vi "UHR-Fleezers Control (host) - Avogadro v2.vi"() -> ()   [LabVIEW 2014] (continued)
      tunnel: w4863 -> [w5493 w5511]
      tunnel: w4862 -> [w5492 w5510]
      tunnel: [w5493 w5506] -> w4814
      tunnel: [w5492 w5505] -> w4813
      tunnel: [FALSE w5504] -> w4846
      tunnel: "Start MCL Scan" -> [_ w5501]
      tunnel: "Confocal Image" -> [_ w5500]
      tunnel: "Confocal Linescan" -> [_ _]
      frame False {
      }
      frame True {
        w5504 = TRUE
        n3101 = case shown="True" "Restart DMA? (MCL)" {
          tunnel: [w5587 w5589] -> w5509
          tunnel: [w5586 w5588] -> w5508
          tunnel: w5511 -> [w5587 w5592]
          tunnel: w5510 -> [w5586 w5591]
          frame False {
          }
          frame True {
            n3102 = call "reset FPGA DMA.vi"("error in"=w5591, "FPGA VI Reference In"=w5592) -> ("error out"=w5588:errorcluster, "FPGA VI Reference Out"=w5589:T40)
            n3103 = local write "Overflow (data lost)"(FALSE ("Overflow (data lost)")) -> ()
          }
        }
        n3104 = case shown="False" w5501 {
          tunnel: w5500 -> [w5514 _]
          frame False {
            n3105 = property on="Confocal Image" class="Bool (strict)"("Value"=FALSE ("Start Confocal Map")) -> ()  [unwired: 2 in, 2 out]
            n3106 = property on="2D or 1D Scan" class="Bool (strict)"("Val(Sgnl)"=w5514) -> ()  [unwired: 2 in, 2 out]
          }
          frame True {
          }
        }
        n3107 = local write "Tab Control 6"(T62."Imaging" ("Tab Control 6")) -> ()
        n3108 = local read "T3 X (V)"() -> (w5496:dbl)
        n3109 = local write "MCL Scanning"(w5504) -> ()
        n3110 = local read "T3 Y (V)"() -> (w5495:dbl)
        n3111 = local read "AO2"() -> (w5497:dbl)
        n3112 = local read "AO1"() -> (w5498:dbl)
        n3113 = case shown="True" "Center Scan" {
          tunnel: w5509 -> [w5527 w5549]
          tunnel: w5508 -> [w5526 w5548]
          tunnel: [w5525 w5547] -> w5506
          tunnel: [w5524 w5546] -> w5505
          tunnel: [w5519 w5543] -> w5503
          tunnel: [w5520 w5542] -> w5502
          tunnel: w5498 -> [w5517 w5545]
          tunnel: w5497 -> [w5516 w5544]
          tunnel: "Scan trap 3 or Fl?" -> [w5522 w5541]
          tunnel: w5496 -> [w5521 w5534]
          tunnel: w5495 -> [w5518 w5535]
          frame False {
            w5523 = TRUE ("AI to FIFO")
            n3114 = case shown="False" w5522 {
              tunnel: [w5529 w5533] -> w5520
              tunnel: w5521 -> [_ w5533]
              tunnel: [w5530 w5532] -> w5519
              tunnel: w5518 -> [_ w5532]
              tunnel: w5517 -> [w5530 _]
              tunnel: w5516 -> [w5529 _]
              tunnel: [FALSE ("AI to FIFO") TRUE ("AI to FIFO")] -> w5515
              frame False {
              }
              frame True {
              }
            }
            n3115 = xnode "Read/Write Control"("FPGA VI Reference In"=w5527, "error in"=w5526, "AI to FIFO"=w5523, "APD to FIFO"=w5523, "Start scan (MCL)"=w5523, "ScanTrap 3 or Fl-laser"=w5515) -> ("FPGA VI Reference Out"=w5525:T40, "error out"=w5524:errorcluster)
          }
          frame True {
            n3116 = local read "Actual MCL Inc (V)"() -> (w5536:dbl)
            n3117 = local read "Scan steps (MCL)"() -> (w5537:u64)
            n3118 = local read "Scan lines (y)"() -> (w5538:u64)
            n3119 = local read "Fast Scan Dir"() -> (w5539:bool)
            n3120 = local read "2D or 1D Scan"() -> (w5540:bool)
            n3121 = case shown="False" w5541 {
              tunnel: w5549 -> [w5567 w5585]
              tunnel: w5548 -> [w5566 w5584]
              tunnel: [w5565 w5583] -> w5547
              tunnel: [w5564 w5582] -> w5546
              tunnel: w5545 -> [w5560 _]
              tunnel: w5544 -> [w5559 _]
              tunnel: [w5557 w5577] -> w5543
              tunnel: [w5556 w5576] -> w5542
              tunnel: w5540 -> [w5555 w5575]
              tunnel: w5539 -> [w5554 w5574]
              tunnel: w5538 -> [w5553 w5573]
              tunnel: w5537 -> [w5552 w5572]
              tunnel: w5536 -> [w5550 w5570]
              tunnel: w5535 -> [_ w5569]
              tunnel: w5534 -> [_ w5568]
              frame False {
                w5563 = TRUE ("AI to FIFO")
                n3122 = Bundle("Actual MCL Inc (V)"=w5550, "Scan steps (MCL)"=w5552, "Scan lines (y)"=w5553, "AO1"=w5560, "AO2"=w5559) -> (w5558:T66)  [unwired: 1 in]
                n3123 = call "Center Scan calculation.vi"("2D or 1D Scan"=w5555, "Fast Scan Dir"=w5554, "Input parameters"=w5558) -> ("X"=w5556:dbl, "Y"=w5557:dbl)
                n3124 = call "Volt to I16.vi"("Voltage In"=w5557) -> ("I16 Voltage Out"=w5562:i16)
                n3125 = call "Volt to I16.vi"("Voltage In"=w5556) -> ("I16 Voltage Out"=w5561:i16)
                n3126 = xnode "Read/Write Control"("FPGA VI Reference In"=w5567, "error in"=w5566, "AI to FIFO"=w5563, "APD to FIFO"=w5563, "Start scan (MCL)"=w5563, "AO1 (Y)"=w5562, "AO2 (X)"=w5561, "ScanTrap 3 or Fl-laser"=FALSE ("AI to FIFO")) -> ("FPGA VI Reference Out"=w5565:T40, "error out"=w5564:errorcluster)
              }
              frame True {
                w5581 = TRUE ("AI to FIFO")
                n3127 = Bundle("Actual MCL Inc (V)"=w5570, "Scan steps (MCL)"=w5572, "Scan lines (y)"=w5573, "T3 Y (V)"=w5569, "T3 X (V)"=w5568) -> (w5578:T67)  [unwired: 1 in]
                n3128 = call "Center Scan calculation.vi"("2D or 1D Scan"=w5575, "Fast Scan Dir"=w5574, "Input parameters"=w5578) -> ("X"=w5576:dbl, "Y"=w5577:dbl)
                n3129 = call "Volt to I16.vi"("Voltage In"=w5577) -> ("I16 Voltage Out"=w5580:i16)
                n3130 = call "Volt to I16.vi"("Voltage In"=w5576) -> ("I16 Voltage Out"=w5579:i16)
                n3131 = xnode "Read/Write Control"("FPGA VI Reference In"=w5585, "error in"=w5584, "AI to FIFO"=w5581, "APD to FIFO"=w5581, "Start scan (MCL)"=w5581, "Piezo Trap Y (AO4)"=w5580, "Piezo Trap X (AO5)"=w5579, "ScanTrap 3 or Fl-laser"=TRUE ("AI to FIFO")) -> ("FPGA VI Reference Out"=w5583:T40, "error out"=w5582:errorcluster)
              }
            }
          }
        }
        "Initial Y" <- w5503
        "Initial X" <- w5502
        "wait to reset values" <- w5504
      }
    }
    n3132 = xnode "Read/Write Control"("FPGA VI Reference In"=w4675) -> ("FPGA VI Reference Out"=w4570:T40, "BD1 Frequency Out 1"=w4677:u64, "Piezo X out"=w4609:i16, "Piezo Y out"=w4608:i16)  [unwired: 1 in, 1 out]
    n3133 = And(x="Save scans", y=w4843) -> (x .and. y?=w4861:bool)
    n3134 = call "IR AOM word to freq.vi"("Frequency Word In (U64)"=w4677) -> ("Frequency Out (MHz)"=w4676:dbl)
    n3135 = Divide(x=w4609, y=w4643) -> (x/y=w4642:dbl)
    n3136 = Divide(x=w4608, y=w4643) -> (x/y=w4641:dbl)
    n3137 = local read "BD 1 Frequency 2 (MHz)"() -> (w4707:dbl)
    n3138 = Subtract(x=w4707, y=w4676) -> (x-y=w4640:dbl)
    "Current deltaF (MHz)" <- w4640
    n3139 = Build Array(w4640, w4642, w4641) -> (w4566:dbl[])
    "Trap position array" <- w4566
    n3140 = control-ref of="Piezo trap cursor control"() -> (w4649:refnum<vi>)
    n3141 = Unbundle By Name("Cursor control") -> ("X"=w4651:bool, "Y"=w4650:bool)
    n3142 = local read "APD Elements/DMA read"() -> (w4738:u32)
    n3143 = local read "Trap AI Elements/DMA read"() -> (w4835:u32)
    n3144 = case shown="False" w4651 {
      tunnel: w4649 -> [w4998 w5008]
      tunnel: w4570 -> [_ w5000]
      frame False {
        n3145 = local read "T3 X (V)"() -> (w4999:dbl)
        n3146 = property class="XYGraph (strict)"(reference=w4998, "Cursor.Cursor X"=w4999) -> ()  [unwired: 1 in, 2 out]
      }
      frame True {
        n3147 = property class="XYGraph (strict)"(reference=w5008) -> ("Cursor.Cursor X"=w5005:dbl)  [unwired: 1 in, 2 out]
        n3148 = In Range and Coerce(upper limit=10.0, x=w5005, lower limit=0.0) -> (coerced(x)=w5003:dbl)  [unwired: 1 out]
        n3149 = Multiply(x=3276.7, y=w5003) -> (x*y=w5002:dbl)
        n3150 = To Unsigned Word Integer(number=w5002) -> (unsigned 16bit integer=w5001:u16)
        n3151 = xnode "Read/Write Control"("FPGA VI Reference In"=w5000, "Piezo Trap X (AO5)"=w5001) -> ()  [unwired: 1 in, 2 out]
      }
    }
    n3152 = case shown="False" w4650 {
      tunnel: w4649 -> [w4985 w4997]
      tunnel: w4570 -> [_ w4988]
      frame False {
        n3153 = local read "T3 Y (V)"() -> (w4987:dbl)
        n3154 = Negate(x=w4987) -> (-x=w4986:dbl)
        n3155 = property class="XYGraph (strict)"(reference=w4985, "Cursor.Cursor Y"=w4986) -> ()  [unwired: 1 in, 2 out]
      }
      frame True {
        n3156 = property class="XYGraph (strict)"(reference=w4997) -> ("Cursor.Cursor Y"=w4994:dbl)  [unwired: 1 in, 2 out]
        n3157 = In Range and Coerce(upper limit=0.0, x=w4994, lower limit=-10.0) -> (coerced(x)=w4993:dbl)  [unwired: 1 out]
        n3158 = Negate(x=w4993) -> (-x=w4991:dbl)
        n3159 = Multiply(x=3276.7, y=w4991) -> (x*y=w4990:dbl)
        n3160 = To Unsigned Word Integer(number=w4990) -> (unsigned 16bit integer=w4989:u16)
        n3161 = xnode "Read/Write Control"("FPGA VI Reference In"=w4988, "Piezo Trap Y (AO4)"=w4989) -> ()  [unwired: 1 in, 2 out]
      }
    }
    n3162 = local read "Trap Pos Elements/DMA read"() -> (w4810:u32)
    n3163 = local read "DMA Update Period (s)"() -> (w4691:dbl)
    n3164 = xnode "Invoke Method"("FPGA VI Reference In"=w4814, "error in"=w4813, "Number of Elements"=w4810, "Timeout (ms)"=-1) -> ("Data"=w4646:u16[], "Elements Remaining"=→"Trap Pos FIFO El Remaining":u32)  [unwired: 2 out]
    n3165 = xnode "Get Trap Data"("FPGA VI Reference In"=w4814, "error in"=w4813, "Number of Elements"=w4835, "Timeout (ms)"=-1 ("Timeout")) -> ("FPGA VI Reference Out"=w4706:T40, "error out"=w4762:errorcluster, "Data"=w4695:i16[], "Elements Remaining"=w4895:u32)
    "FIFO El. Rem." <- w4895
    n3166 = local read "Trap AI FIFO Depth"() -> (w4897:u32)
    n3167 = xnode "Get APD Data"("FPGA VI Reference In"=w4814, "error in"=w4813, "Number of Elements"=w4738, "Timeout (ms)"=-1) -> ("Data"=w4687:u32[], "Elements Remaining"=→"APD FIFO Elements Remaining":u32)  [unwired: 2 out]
    n3168 = feedback #1(0.0) -> (w4808:dbl)
    n3169 = To Time Stamp(1:w4808) -> (0:w4590:timestamp)
    n3170 = Add(x=w4691, y=w4808) -> (x+y=w4872:dbl)
    n3171 = feedback-in #1(w4872) -> ()
    n3172 = Subtract(x=w4897, y=w4835) -> (x-y=w4896:u32)
    n3173 = local read "APD Integration Time (s)"() -> (w4679:dbl)
    n3174 = Divide(x=w4895, y=w4896) -> (x/y=w4894:dbl)
    "Buffer Status" <- w4894
    n3175 = local read "Trap Sets"() -> (w4696:u32)
    n3176 = Equal?(x=w4894, y=1.0) -> (x = y?=w4892:bool)
    n3177 = local read "Number of APDs"() -> (w4686:u8)
    n3178 = case "Alert buffer overflow" shown="True" w4892 {
      frame False {
      }
      frame True {
        n3179 = call <vilib>:"Beep.vi"() -> ()  [unwired: 3 in, 9 out]
        "Overflow (data lost)" <- TRUE ("Overflow (data lost)")
      }
    }
    n3180 = call "deinterlace.vi"("Detector type"="Detector Type", "Data"=w4695, "Trap sets"=w4696, "Flip x sign"="Flip X Sign") -> ("Channel pattern"=w4692:i32, "Channel names"=w4648:string[], "Deinterlaced normalized data"=w4584:dbl[][], "Deinterlaced data"=w4693:i16[])
    "AI labels" <- w4648
    n3181 = local read "Data Period (s)"() -> (w4583:dbl)
    n3182 = call "Trap_position_vectors.vi"("Data array"=w4646) -> ("Output data for plotting"=w4645:dbl[][], "Output data for saving"=w4644:u64[])
    n3183 = call "APD data extraction.vi"("Data"=w4687, "Number of APD's"=w4686, "APD integration time (s)"=w4679, "APD Ave N"="APD Ave N", "APD Disp. Downsample"="APD Disp. Downsample", "APD Disp. Scale"="APD Disp. Scale", "Time Stamp"=w4590) -> ("Output cluster"=→"APD rates cluster":T2, "Output Data"=w4682:T68, "Output waveform"=w4681:waveform(dbl)[], "APD Display period (s)"=w4680:dbl)
    "APD Display Period (s)" <- w4680
    n3184 = Reciprocal(x=w4680) -> (1/x=→"APD Display Freq. (Hz)":dbl)
    n3185 = Multiply(x=w4583, y="Trap Disp. Downsample") -> (x*y=w4809:dbl)
    "Display Period (s)" <- w4809
    n3186 = for {
      tunnel: w4584 -> [w5023] mode=indexing
      tunnel: [w5022] -> w4647 mode=indexing
      n3187 = call-poly <vilib>:"Mean.vi"("X"=w5023) -> ("mean"=w5022:dbl)  [unwired: 1 out]
    }
    "Values" <- w4647
    n3188 = Decimate 1D Array(w4693) -> (w4800:i16[], w4799:i16[], w4797:i16[], w4796:i16[])  [unwired: 9 out]
    n3189 = call "Generate Waveform.vi"("Downsampling"="Trap Disp. Downsample", "Data Period (s)"=w4583, "Data"=w4584, "Plot names"=w4648, "Time Stamp"=w4590) -> ("Downsampled data"=w4626:waveform(dbl)[], "Non downsampled waveform"=w4688:waveform(dbl)[])
    n3190 = Multiply(x="APD Disp. Scale", y=w4681) -> (x*y=w4818:waveform(dbl)[])
    n3191 = Reciprocal(x=w4809) -> (1/x=→"Trap Disp. Freq. (Hz)":dbl)
    n3192 = Multiply(x="APD Disp. Downsample", y=w4679) -> (x*y=w4817:dbl)
    n3193 = Divide(x=w4800, y=w4799) -> (x/y=w4801:dbl[])
    n3194 = Divide(x=w4797, y=w4796) -> (x/y=w4798:dbl[])
    n3195 = Divide(x=w4818, y=w4817) -> (x/y=w4742:waveform(dbl)[])
    n3196 = case shown="1" "Plot Trap Positions" {
      tunnel: [w5009 w5017] -> w4670
      frame 0, Default {
        n3197 = local read "BD 1 Frequency 2 (MHz)"() -> (w5012:dbl)
        n3198 = local read "BD 1 Frequency 1 (MHz)"() -> (w5013:dbl)
        n3199 = local read "T3 Y (V)"() -> (w5010:dbl)
        n3200 = local read "T3 X (V)"() -> (w5011:dbl)
        n3201 = Build Array(w5013, w5012, w5011, w5010) -> (w5009:dbl[])
      }
      frame 1 {
        w5016 = 60.0
        n3202 = local read "Piezo trap x\noffset (V)"() -> (w5014:dbl)
        n3203 = Build Array(w5016, w5016, w5014, "Piezo trap y\noffset (V)") -> (w5017:dbl[])
      }
    }
    n3204 = Split 1D Array(array=w4801, index="N El. to Ave.") -> (second subarray=w4804:dbl[])  [unwired: 1 out]
    n3205 = Split 1D Array(array=w4798, index="N El. to Ave.") -> (second subarray=w4803:dbl[])  [unwired: 1 out]
    n3206 = case shown="True" "Chart APD?" {
      tunnel: w4742 -> [_ w4963]
      frame False {
      }
      frame True {
        n3207 = Index Array(array=w4963, index=0) -> (element=w4973:waveform(dbl))
        n3208 = Index Array(array=w4963, index=1) -> (element=w4971:waveform(dbl))
        n3209 = Index Array(array=w4963, index=2) -> (element=w4965:waveform(dbl))
        n3210 = Subtract(x=w4973, y="APD 1 Offset") -> (x-y=w4969:waveform(dbl))
        n3211 = Subtract(x=w4971, y="APD 2 Offset") -> (x-y=w4968:waveform(dbl))
        n3212 = Subtract(x=w4965, y="APD 3 Offset") -> (x-y=w4962:waveform(dbl))
        n3213 = Build Array(w4969, w4968, w4962) -> (→"APD Chart":waveform(dbl)[])
      }
    }
    n3214 = local read "AOM X Cal (nm/MHz)"() -> (w4672:dbl)
    n3215 = call-poly <vilib>:"Mean.vi"("X"=w4804) -> ("mean"=w4792:dbl)  [unwired: 1 out]
    n3216 = call-poly <vilib>:"Mean.vi"("X"=w4803) -> ("mean"=w4791:dbl)  [unwired: 1 out]
    n3217 = local read "Trap X AI1 (DMA)"() -> (w4802:T23)
    n3218 = To Fixed-Point(number=w4791) -> (fixed-point=w4789:fxp<+/-,16,1>)  [unwired: 1 in]
    n3219 = To Fixed-Point(number=w4792) -> (fixed-point=w4790:fxp<+/-,16,1>)  [unwired: 1 in]
    n3220 = Bundle By Name(cluster=w4802, "Set 1"=w4790, "Set 2"=w4789) -> (→"Trap X AI1 (DMA)":T23)
    n3221 = Build Array(w4672, w4672, "Piezo Trap X cal (nm/V)", "Piezo Trap Y cal (nm/V)") -> (w4671:dbl[])
    n3222 = Cluster To Array(cluster="Negate Axis") -> (array=w4665:bool[])
    n3223 = call "Generate Trap Positiion Waveform.vi"("Base trap positions"=w4670, "Data Period (s)"=w4583, "Input data"=w4645, "Position calibration values"=w4671, "Trap Pos. Disp. Downsample (s)"="Trap Pos. Disp. Downsample", "Negate axis"=w4665, "Time Stamp"=w4590) -> ("Output waveforms"=w4653:waveform(dbl)[], "Output trap positions"=w4599:cluster{"X":dbl[], "Y":dbl[]}[])  [unwired: 2 in]
    "Trap Positions" <- w4653
    n3224 = Initialize Array(0.0) -> (w4667:dbl[][])  [unwired: 2 in]
    n3225 = local read "Display Period (s)"() -> (w4826:dbl)
    n3226 = for {
      tunnel: w4653 -> [w5021] mode=indexing
      shift-right: [w5019] -> w4655
      shift-left: w4667 -> [w5020]
      n3227 = Unbundle By Name(w5021) -> ("Y"=w5018:dbl[])
      n3228 = Build Array (concatenate)(w5020, w5018) -> (w5019:dbl[][])
    }
    n3229 = Build Array (concatenate)(w4681, w4626) -> (w4690:waveform(dbl)[])
    "All Signals" <- w4690
    n3230 = Initialize Array(0.0) -> (w4580:dbl[][])  [unwired: 2 in]
    n3231 = feedback #2(w4580) -> (w4579:dbl[][])
    n3232 = Divide(x="Bead Sep. Int. Time (s)", y=w4826) -> (x/y=w4661:dbl)
    n3233 = case shown="True" "Start position \nscan" {
      tunnel: w4579 -> [w4976 _]
      tunnel: [w4976 w4984] -> w4578
      tunnel: "T3 positioning test range (V)" -> [_ w4978]
      frame False {
      }
      frame True {
        n3234 = local read "BD 1 Frequency 1 (MHz)"() -> (→"AOM position for scan (MHz)":dbl)
        n3235 = Unbundle By Name(w4978) -> ("Xmin"=w4980:dbl, "Ymin"=w4979:dbl)
        n3236 = local write "Start position \nscan"(FALSE) -> ()
        n3237 = local write "T3 X (V)"(w4980) -> ()
        n3238 = local write "T3 Y (V)"(w4979) -> ()
        n3239 = Initialize Array(0.0) -> (w4984:dbl[][])  [unwired: 2 in]
        "Position\nscanning..." <- TRUE
      }
    }
    n3240 = case shown="True" "Measure \ncorrelation?" {
      tunnel: w4584 -> [_ w4950]
      tunnel: w4583 -> [_ w4949]
      tunnel: w4578 -> [w4920 w4933]
      tunnel: [w4920 w4926] -> w4577
      tunnel: "T3 positioning test range (V)" -> [_ w4925]
      tunnel: w4570 -> [_ w4921]
      frame False {
      }
      frame True {
        n3241 = local read "DMA Update Period (s)"() -> (w4928:dbl)
        n3242 = Divide(x="Correlation integration time (s)", y=w4928) -> (x/y=w4927:dbl)
        n3243 = To Word Integer(number=w4927) -> (16bit integer=w4923:i16)
        n3244 = Divide(x="Correlation integration time (s)", y=w4949) -> (x/y=w4943:dbl)
        n3245 = Initialize Array(0.0, w4943, 4) -> (w4946:dbl[][])
        n3246 = feedback #3(w4946) -> (w4945:dbl[][])
        n3247 = call "correlation calculation for trap 3 absolute positioning.vi"("Number of sets to average"=w4943, "Accumulated array"=w4945, "raw data"=w4950) -> ("Accumulated array out"=w4944:dbl[][], "Y correlation"=w4941:dbl, "X correlation"=w4942:dbl)
        "3-1 x correlation" <- w4942
        "3-1 y correlation" <- w4941
        n3248 = feedback-in #3(w4944) -> ()
        n3249 = Increment(x=w4923) -> (x+1=w4922:i16)
        n3250 = local read "Position\nscanning..."() -> (w4932:bool)
        n3251 = Bundle("X correlation"=w4942, "Y correlation"=w4941) -> (w4940:T69)  [unwired: 1 in]
        n3252 = local read "T3 Y (V)"() -> (w4938:dbl)
        n3253 = local read "T3 X (V)"() -> (w4939:dbl)
        n3254 = Bundle("T3 X (V)"=w4939, "T3 Y (V)"=w4938) -> (w4937:cluster{"T3 X (V)":dbl, "T3 Y (V)":dbl})  [unwired: 1 in]
        n3255 = feedback #4(i16 0) -> (w4935:i16)
        n3256 = call "correlation scan.vi"("Correlations in"=w4940, "Voltages in"=w4937, "Cycle counter"=w4935, "in put Array"=w4933, "T3 positioning \ntest range (V)"=w4925, "Number of acquisition cycles"=w4922, "Scanning?"=w4932) -> ("Voltages out"=w4930:cluster{"X":dbl, "Y":dbl}, "Scanning out"=w4931:bool, "Output array"=w4926:dbl[][], "Cycle counter out"=w4934:i16)
        n3257 = feedback-in #4(w4934) -> ()
        n3258 = local write "Position\nscanning..."(w4931) -> ()
        n3259 = case shown="True" w4931 {
          tunnel: w4930 -> [_ w4961]
          tunnel: w4921 -> [_ w4955]
          frame False {
          }
          frame True {
            w4959 = 3276.7
            n3260 = Unbundle By Name(w4961) -> ("X"=w4960:dbl, "Y"=w4958:dbl)
            n3261 = Multiply(x=w4959, y=w4960) -> (x*y=w4957:dbl)
            n3262 = Multiply(x=w4959, y=w4958) -> (x*y=w4956:dbl)
            n3263 = To Word Integer(number=w4957) -> (16bit integer=w4954:i16)
            n3264 = To Word Integer(number=w4956) -> (16bit integer=w4953:i16)
            n3265 = local write "T3 Y (V)"(w4958) -> ()
            n3266 = local write "T3 X (V)"(w4960) -> ()
            n3267 = xnode "Read/Write Control"("FPGA VI Reference In"=w4955, "Piezo Trap X (AO5)"=w4954, "Piezo Trap Y (AO4)"=w4953) -> ()  [unwired: 1 in, 2 out]
          }
        }
        n3268 = case shown="True" "Stop scan" {
          frame False {
          }
          frame True {
            n3269 = local write "Position\nscanning..."(FALSE) -> ()
            n3270 = local write "Stop scan"(FALSE) -> ()
          }
        }
      }
    }
    n3271 = feedback-in #2(w4577) -> ()
    n3272 = feedback #5(w4655) -> (w4662:dbl[][])
    n3273 = call "Trap Pos RMS.vi"("Accumulated array"=w4662, "New Array"=w4655, "Number of sets to average"=w4661) -> ("Output accumulated array"=w4660:dbl[][], "RMS"=w4658:dbl[], "Mean"=w4659:dbl[])
    n3274 = feedback-in #5(w4660) -> ()
    n3275 = Index Array(array=w4655, index (row)=0 ("index")) -> (element=w4654:dbl[])  [unwired: 1 in]
    n3276 = local read "Two Trap Offset Values"() -> (w4636:T31)
    n3277 = Array To Cluster(array=w4658) -> (cluster=→"Trap RMS (ang)":T70)
    n3278 = Array To Cluster(array=w4659) -> (cluster=→"Mean Trap Positions (nm)":T71)
    n3279 = local read "MCL offset scanning range (V)"() -> (w4634:T4)
    n3280 = local read "Multi-MCL offset array"() -> (w4635:T30)
    n3281 = local read "Multiple-MCL offset?"() -> (w4639:bool)
    n3282 = local read "Offset file step size"() -> (w4637:dbl)
    n3283 = local read "T1 calibration"() -> (w4633:T12)
    n3284 = local read "T2 calibration"() -> (w4632:T12)
    n3285 = local read "T3 calibration"() -> (w4631:T12)
    n3286 = local read "Trap Disp. Downsample"() -> (w4588:dbl)
    n3287 = Build Array(w4633, w4632, w4631) -> (w4630:T55)
    n3288 = call "calibrate trap data V3RG.vi"("array of calibration clusters"=w4630, "Trap position array"=w4566, "MCL offset scanning range (V)"=w4634, "Multi-MCL offset array"=w4635, "two trap offset values"=w4636, "Dynamic offset update"="Dynamic offset\nupdate", "Multiple-MCL offset?"=w4639, "x (true) or y (false)"=TRUE, "Data array"=w4626, "Offset File step size"=w4637) -> ("Positions out"=w4628:dbl[][], "Forces out (pN)"=w4627:dbl[][])
    n3289 = local read "Mean Trap Positions (nm)"() -> (w4625:T6)
    n3290 = local read "Trap 2 Bead Size (nm)"() -> (w4603:dbl)
    n3291 = local read "Trap 3 Bead Size (nm)"() -> (w4602:dbl)
    n3292 = local read "Trap 1 Bead Size (nm)"() -> (w4604:dbl)
    n3293 = case shown="True" "Measure \ncorrelation?" {
      tunnel: w4577 -> [_ w4904]
      tunnel: "T3 positioning test range (V)" -> [_ w4903]
      frame False {
      }
      frame True {
        n3294 = Unbundle By Name(w4903) -> ("Xmax"=w4907:dbl, "Xmin"=w4908:dbl, "increment"=w4913:dbl, "Ymax"=w4909:dbl, "Ymin"=w4910:dbl)
        n3295 = Index Array(array=w4904, index (col)=3) -> (element=w4906:dbl[])  [unwired: 1 in]
        n3296 = Index Array(array=w4904, index (col)=2) -> (element=w4905:dbl[])  [unwired: 1 in]
        n3297 = Subtract(x=w4909, y=w4910) -> (x-y=w4912:dbl)
        n3298 = Subtract(x=w4907, y=w4908) -> (x-y=w4911:dbl)
        n3299 = Quotient & Remainder(x=w4912, y=w4913) -> (floor(x/y)=w4915:dbl)  [unwired: 1 out]
        n3300 = Quotient & Remainder(x=w4911, y=w4913) -> (floor(x/y)=w4914:dbl)  [unwired: 1 out]
        n3301 = Increment(x=w4914) -> (x+1=w4917:dbl)
        n3302 = Increment(x=w4915) -> (x+1=w4916:dbl)
        n3303 = Reshape Array(w4906, w4917, w4916) -> (→"Correlations in Y":dbl[][])
        n3304 = Reshape Array(w4905, w4917, w4916) -> (→"Correlations in X":dbl[][])
      }
    }
    n3305 = local read "Data Period (s)"() -> (w4592:dbl)
    n3306 = Index Array(array=w4626, index="index 2") -> (element=w4737:waveform(dbl))
    n3307 = Index Array(array=w4626, index="index 1") -> (element=w4733:waveform(dbl))
    n3308 = Multiply(x=w4588, y=w4592) -> (x*y=w4591:dbl)
    n3309 = Unbundle By Name(w4737) -> ("Y"=w4736:dbl[])
    n3310 = Unbundle By Name(w4733) -> ("Y"=w4732:dbl[])
    n3311 = Build Array(w4604, w4603, w4602) -> (w4601:dbl[])
    n3312 = call "Force and position waveforms.vi"("Input waveforms"=w4626, "Forces  (pN)"=w4627, "Deflections (nm)"=w4628, "Mean Trap Positions (nm)"=w4625) -> ("1D data"=w4611:waveform(dbl)[], "Absolute Positions"=w4607:waveform(dbl)[], "Forces"=w4585:waveform(dbl)[], "Deflections"=w4606:waveform(dbl)[], "Raw Data"=w4605:waveform(dbl)[])
    n3313 = call-poly <vilib>:"Mean.vi"("X"=w4732) -> ("mean"=→"Trap 1 sum mean":dbl)  [unwired: 1 out]
    n3314 = call-poly <vilib>:"Mean.vi"("X"=w4736) -> ("mean"=→"Trap 2 sum mean":dbl)  [unwired: 1 out]
    n3315 = local read "Trap 3 Bead Size (nm)"() -> (w4575:dbl)
    n3316 = call "2D force plotting.vi"("Trap positions"=w4599, "Calibration"="2D force calibration", "Bead sizes"=w4601, "Raw Data"=w4605, "Deflections"=w4606, "Forces"=w4585, "Absolute Positions"=w4607) -> ("Output waveforms"=→"2D forces":waveform(dbl)[], "Output"=→"2D values (force/position/raw)":T1, "Junctions"=w4597:cluster{"X":dbl[], "Y":dbl[]}[], "deflection lines"=w4598:cluster{"X":dbl[], "Y":dbl[]}[], "tether sizes"=w4593:dbl[][])
    n3317 = local read "Trap 2 Bead Size (nm)"() -> (w4613:dbl)
    n3318 = local read "Trap 1 Bead Size (nm)"() -> (w4614:dbl)
    n3319 = call "2D tether waveforms.vi"("tether sizes"=w4593, "Data period (s)"=w4591, "Time Stamp"=w4590, "Forces"=w4585) -> ("tethers"=→"2D tethers":waveform(dbl)[], "output forces"=→"tether forces":waveform(dbl)[], "Output Means"=→"Output Means":T9)  [unwired: 2 in]
    n3320 = call "1D force plotting.vi"("Calibration"="Calibration", "Forces"=w4585, "Deflections"=w4606, "Raw Data"=w4605, "Only check fixed trap T2"="Only check fixed trap T2") -> ("Vec Mean of T1 T2"=→"Vec Mean of T1 T2":dbl[], "Output force values"=w4620:T72, "Output waveforms"=→"Force":waveform(dbl)[])
    n3321 = call "1D bead separation calculation.vi"("Trap 1 Bead Size (nm)"=w4614, "Trap 2 Bead Size (nm)"=w4613, "Trap 3 Bead Size (nm)"=w4575, "Absolute Positions"=w4607, "Pair choice"="Pair to \nanalyze") -> ("Output separation"=w4612:dbl[], "Output waveforms"=w4572:waveform(dbl)[])
    "Bead Separation" <- w4572
    n3322 = Build Array (concatenate)(w4599, w4598, w4597) -> (→"Positions \nand displacements":cluster{"X":dbl[], "Y":dbl[]}[])
    n3323 = Unbundle By Name(w4620) -> ("T1 X"=→"T1 X":dbl, "T2 X"=→"T2 X":dbl, "Mean"=w4617:dbl, "Difference"=→"Difference":dbl)
    "Mean" <- w4617
    n3324 = Subtract(x=w4612, y="Offset (nm)") -> (x-y=w4829:dbl[])
    n3325 = feedback #6(w4829) -> (w4828:dbl[])
    n3326 = Build Array (concatenate)(w4829, w4828) -> (w4721:dbl[])
    n3327 = Split 1D Array(array=w4721, index=w4661) -> (first subarray=w4722:dbl[])  [unwired: 1 out]
    n3328 = feedback-in #6(w4722) -> ()
    n3329 = Index Array(array=w4572, index=0) -> (element=w4571:waveform(dbl))
    n3330 = call-poly <vilib>:"Mean.vi"("X"=w4722) -> ("mean"=w4825:dbl)  [unwired: 1 out]
    "Bead Mean (nm)" <- w4825
    n3331 = Build Array (concatenate)(w4611, w4571) -> (w4624:waveform(dbl)[])
    n3332 = Subtract(x=w4722, y=w4825) -> (x-y=w4824:dbl[])
    n3333 = Square(x=w4824) -> (x^2=w4823:dbl[])
    n3334 = call-poly <vilib>:"Mean.vi"("X"=w4823) -> ("mean"=w4822:dbl)  [unwired: 1 out]
    n3335 = Square Root(x=w4822) -> (sqrt(x)=w4821:dbl)
    n3336 = Multiply(x=10.0, y=w4821) -> (x*y=→"RMS (Ang)":dbl)
    n3337 = local read "Data points/scans (MCL)"() -> (w4855:dbl)
    n3338 = Unbundle(w4682) -> ("APD 1"=w4741:u32[])  [unwired: 2 out]
    n3339 = To Double Precision Float(number=w4741) -> (double precision float=w4830:dbl[])
    n3340 = Increment(x=w4855) -> (x+1=w4856:dbl)
    n3341 = feedback #7(w4856) -> (w4859:dbl)
    n3342 = Select(t=0, s=w4846, f=w4859) -> (s? t:f=w4852:dbl)
    n3343 = Array Size(array=w4830) -> (size(s)=w4858:i32)
    n3344 = Add(x=w4858, y=w4852) -> (x+y=w4853:dbl)
    n3345 = Greater?(x=w4853, y=w4855) -> (0:w4854:bool)
    n3346 = local read "MCL Scanning"() -> (w4849:bool)
    n3347 = Select(t=w4852, s=w4854, f=w4853) -> (s? t:f=w4851:dbl)
    n3348 = feedback-in #7(w4851) -> ()
    n3349 = Not(x=w4854) -> (.not. x?=w4848:bool)
    n3350 = And(x=w4848, y=w4849) -> (x .and. y?=w4850:bool)
    n3351 = Or(x=w4850, y=w4846) -> (x .or. y?=w4847:bool)
    n3352 = Equal?(x="Tab Control 6", y=T61."High Res Display") -> (x = y?=w4832:bool)
    n3353 = case "For displaying the high resolution display (no downsampling)" shown="True" w4832 {
      tunnel: w4688 -> [_ w5276]
      frame False {
      }
      frame True {
        n3354 = Index Array(array=w5276, index="High Res. Display") -> (element=w5277:waveform(dbl))
        n3355 = call <vilib>:"Std Deviation and Variance.vi"("X"=w5277) -> ("mean"=w5284:dbl, "standard deviation"=w5289:dbl)  [unwired: 1 in, 1 out]
        "Mean Intensity" <- w5284
        "Sigma" <- w5289
        n3356 = Subtract(x=w5277, y=w5284) -> (x-y=w5283:waveform(dbl))
        n3357 = Select(t=w5283, s="Subtract mean", f=w5277) -> (s? t:f=→"1 Channel":waveform(dbl))
        n3358 = Divide(x=w5289, y=w5284) -> (x/y=→"Sigma/Mean":dbl)
        n3359 = feedback #8(1) -> (w5278:i32)
        n3360 = Greater Or Equal?(x=w5278, y="Slow mean N ave.") -> (x >= y?=w5291:bool)
        n3361 = Increment(x=w5278) -> (x+1=w5293:i32)
        n3362 = Select(t=1, s=w5291, f=w5293) -> (s? t:f=w5280:i32)
        n3363 = feedback-in #8(w5280) -> ()
        n3364 = feedback #9() -> (w5281:waveform(dbl))  [unwired: 1 out]
        n3365 = case shown="Default" w5278 {
          tunnel: [w5296 w5299] -> w5282
          tunnel: w5281 -> [w5298 _]
          tunnel: w5277 -> [w5297 w5299]
          frame Default {
            n3366 = call-poly <vilib>:"Append Waveforms.vi"("waveform B"=w5297, "waveform A"=w5298) -> ("waveform out"=w5296:waveform(dbl))  [unwired: 1 in, 8 out]
          }
          frame 1 {
          }
        }
        n3367 = feedback-in #9(w5282) -> ()
        n3368 = case shown="True" w5291 {
          tunnel: w5282 -> [_ w5295]
          frame False {
          }
          frame True {
            n3369 = call-poly <vilib>:"Mean.vi"("X"=w5295) -> ("mean"=→"Slow mean":dbl)  [unwired: 1 out]
          }
        }
      }
    }
    n3370 = case "For plotting results of scanning MCL (fluorescence and detection laser images)" shown="True" w4847 {
      tunnel: w4846 -> [_ w5353]
      tunnel: w4855 -> [_ _]
      tunnel: w4688 -> [_ w5449]
      tunnel: w4815 -> [_ w5381]
      tunnel: w4682 -> [_ w5359]
      frame False {
      }
      frame True {
        # "Modified by Ronen \nbecause we do not have\nthe license for the\ntwo last image \nmanipulation VI's"
        n3371 = local read "Scan trap 3 or Fl?"() -> (w5337:bool)
        n3372 = case shown="True" w5337 {
          tunnel: [10 ("index") 0 ("index")] -> w5456
          tunnel: [11 ("index") 1 ("index")] -> w5453
          frame False {
          }
          frame True {
          }
        }
        n3373 = Unbundle(w5359) -> ("APD 1"=w5358:u32[], "APD 2"=w5356:u32[], "APD 3"=w5354:u32[])
        n3374 = To Double Precision Float(number=w5358) -> (double precision float=w5357:dbl[])
        n3375 = To Double Precision Float(number=w5356) -> (double precision float=w5355:dbl[])
        n3376 = To Double Precision Float(number=w5354) -> (double precision float=w5347:dbl[])
        n3377 = Index Array(array=w5449, index=w5456) -> (element=w5455:waveform(dbl))
        n3378 = Index Array(array=w5449, index=w5453) -> (element=w5452:waveform(dbl))
        n3379 = local read "Cycles/step (MCL)"() -> (w5411:u64)
        n3380 = Index Array(array=w5449, index="Channel") -> (element=w5451:waveform(dbl))
        n3381 = Unbundle(w5381) -> ("New Image"=w5380:T8, "New Image"=w5379:T8, "New Image"=w5360:T8, "New Image"=w5361:T8, "New Image"=w5362:T8)
        n3382 = local read "Scan steps (MCL)"() -> (w5349:u64)
        n3383 = Unbundle By Name(w5455) -> ("Y"=w5413:dbl[])
        n3384 = Unbundle By Name(w5452) -> ("Y"=w5415:dbl[])
        n3385 = local read "Scan lines (y)"() -> (w5350:u64)
        n3386 = local read "N APD Samp/step"() -> (w5352:dbl)
        n3387 = Unbundle By Name(w5451) -> ("Y"=w5420:dbl[])
        n3388 = call "downsample 1D array - double.vi"("Ave N"=w5411, "Array In"=w5413) -> ("Array Out"=w5412:dbl[])  [unwired: 1 out]
        n3389 = call "downsample 1D array - double.vi"("Ave N"=w5411, "Array In"=w5415) -> ("Array Out"=w5414:dbl[])  [unwired: 1 out]
        n3390 = call "downsample 1D array - double.vi"("Ave N"=w5411, "Array In"=w5420) -> ("Array Out"=w5419:dbl[])  [unwired: 1 out]
        n3391 = Multiply(x=w5349, y=u64 2) -> (x*y=w5351:u64)
        n3392 = feedback #10(w5355) -> (w5399:dbl[])
        n3393 = Build Array (concatenate)(w5399, w5355) -> (w5398:dbl[])
        n3394 = feedback #11(w5347) -> (w5348:dbl[])
        n3395 = Build Array (concatenate)(w5348, w5347) -> (w5346:dbl[])
        n3396 = Select(t=w5355, s=w5353, f=w5398) -> (s? t:f=w5383:dbl[])
        n3397 = feedback-in #10(w5383) -> ()
        n3398 = Select(t=w5347, s=w5353, f=w5346) -> (s? t:f=w5364:dbl[])
        n3399 = feedback-in #11(w5364) -> ()
        n3400 = feedback #12(w5357) -> (w5474:dbl[])
        n3401 = Build Array (concatenate)(w5474, w5357) -> (w5457:dbl[])
        n3402 = Select(t=w5357, s=w5353, f=w5457) -> (s? t:f=w5461:dbl[])
        n3403 = feedback-in #12(w5461) -> ()
        n3404 = feedback #13(w5412) -> (w5463:dbl[])
        n3405 = Build Array (concatenate)(w5463, w5412) -> (w5454:dbl[])
        n3406 = feedback #14(w5419) -> (w5472:dbl[])
        n3407 = Build Array (concatenate)(w5472, w5419) -> (w5471:dbl[])
        n3408 = feedback #15(w5414) -> (w5465:dbl[])
        n3409 = Build Array (concatenate)(w5465, w5414) -> (w5466:dbl[])
        n3410 = Select(t=w5412, s=w5353, f=w5454) -> (s? t:f=w5416:dbl[])
        n3411 = feedback-in #13(w5416) -> ()
        n3412 = Select(t=w5419, s=w5353, f=w5471) -> (s? t:f=w5418:dbl[])
        n3413 = feedback-in #14(w5418) -> ()
        n3414 = Select(t=w5414, s=w5353, f=w5466) -> (s? t:f=w5417:dbl[])
        n3415 = feedback-in #15(w5417) -> ()
        n3416 = call "integrate 1D array interval - double.vi"("Ave N"=w5352, "Array In"=w5383) -> ("Array Out"=w5394:dbl[])  [unwired: 1 out]
        n3417 = call "integrate 1D array interval - double.vi"("Ave N"=w5352, "Array In"=w5364) -> ("Array Out"=w5375:dbl[])  [unwired: 1 out]
        n3418 = call "integrate 1D array interval - double.vi"("Ave N"=w5352, "Array In"=w5461) -> ("Array Out"=w5460:dbl[])  [unwired: 1 out]
        n3419 = Array Size(array=w5394) -> (size(s)=w5395:i32)
        n3420 = Array Size(array=w5375) -> (size(s)=w5376:i32)
        n3421 = Array Size(array=w5460) -> (size(s)=w5462:i32)
        n3422 = Multiply(x=w5350, y=w5351) -> (x*y=w5397:u64)
        n3423 = Multiply(x=w5350, y=w5351) -> (x*y=w5378:u64)
        n3424 = Multiply(x=w5350, y=w5351) -> (x*y=w5470:u64)
        n3425 = Subtract(x=w5397, y=w5395) -> (x-y=w5388:u64)
        n3426 = call-poly <vilib>:"Mean.vi"("X"=w5394) -> ("mean"=w5385:dbl)  [unwired: 1 out]
        n3427 = Subtract(x=w5378, y=w5376) -> (x-y=w5369:u64)
        n3428 = call-poly <vilib>:"Mean.vi"("X"=w5375) -> ("mean"=w5366:dbl)  [unwired: 1 out]
        n3429 = Subtract(x=w5470, y=w5462) -> (x-y=w5410:u64)
        n3430 = call-poly <vilib>:"Mean.vi"("X"=w5460) -> ("mean"=w5407:dbl)  [unwired: 1 out]
        n3431 = call-poly <vilib>:"Mean.vi"("X"=w5416) -> ("mean"=w5400:dbl)  [unwired: 1 out]
        n3432 = call-poly <vilib>:"Mean.vi"("X"=w5418) -> ("mean"=w5405:dbl)  [unwired: 1 out]
        n3433 = call-poly <vilib>:"Mean.vi"("X"=w5417) -> ("mean"=w5403:dbl)  [unwired: 1 out]
        n3434 = Initialize Array(1.0 ("element"), w5388) -> (w5384:dbl[])
        n3435 = Initialize Array(1.0 ("element"), w5369) -> (w5365:dbl[])
        n3436 = Initialize Array(1.0 ("element"), w5410) -> (w5401:dbl[])
        n3437 = Multiply(x=w5384, y=w5385) -> (x*y=w5386:dbl[])
        n3438 = Multiply(x=w5365, y=w5366) -> (x*y=w5367:dbl[])
        n3439 = Multiply(x=w5401, y=w5407) -> (x*y=w5408:dbl[])
        n3440 = Multiply(x=w5401, y=w5403) -> (x*y=w5404:dbl[])
        n3441 = Multiply(x=w5401, y=w5405) -> (x*y=w5406:dbl[])
        n3442 = Multiply(x=w5401, y=w5400) -> (x*y=w5402:dbl[])
        n3443 = Build Array (concatenate)(w5394, w5386) -> (w5396:dbl[])
        n3444 = Build Array (concatenate)(w5375, w5367) -> (w5377:dbl[])
        n3445 = Build Array (concatenate)(w5460, w5408) -> (w5469:dbl[])
        n3446 = Build Array (concatenate)(w5416, w5402) -> (w5464:dbl[])
        n3447 = Build Array (concatenate)(w5418, w5406) -> (w5468:dbl[])
        n3448 = Build Array (concatenate)(w5417, w5404) -> (w5467:dbl[])
        n3449 = Reshape Array(w5396, w5350, w5351) -> (w5392:dbl[][])
        n3450 = Reshape Array(w5377, w5350, w5351) -> (w5373:dbl[][])
        n3451 = Reshape Array(w5469, w5350, w5351) -> (w5447:dbl[][])
        n3452 = Reshape Array(w5464, w5350, w5351) -> (w5430:dbl[][])
        n3453 = Reshape Array(w5468, w5350, w5351) -> (w5422:dbl[][])
        n3454 = Reshape Array(w5467, w5350, w5351) -> (w5437:dbl[][])
        n3455 = Array Subset(array=w5392, index (col)=0 ("index"), length (col)=w5349) -> (w5391:dbl[][])  [unwired: 2 in]
        n3456 = Array Subset(array=w5392, index (col)=w5349) -> (w5389:dbl[][])  [unwired: 3 in]
        n3457 = Array Subset(array=w5373, index (col)=0 ("index"), length (col)=w5349) -> (w5372:dbl[][])  [unwired: 2 in]
        n3458 = Array Subset(array=w5373, index (col)=w5349) -> (w5370:dbl[][])  [unwired: 3 in]
        n3459 = Array Subset(array=w5437, index (col)=0 ("index"), length (col)=w5349) -> (w5442:dbl[][])  [unwired: 2 in]
        n3460 = Array Subset(array=w5437, index (col)=w5349) -> (w5440:dbl[][])  [unwired: 3 in]
        n3461 = Array Subset(array=w5447, index (col)=0 ("index"), length (col)=w5349) -> (w5446:dbl[][])  [unwired: 2 in]
        n3462 = Array Subset(array=w5447, index (col)=w5349) -> (w5444:dbl[][])  [unwired: 3 in]
        n3463 = Array Subset(array=w5422, index (col)=0 ("index"), length (col)=w5349) -> (w5428:dbl[][])  [unwired: 2 in]
        n3464 = Array Subset(array=w5422, index (col)=w5349) -> (w5426:dbl[][])  [unwired: 3 in]
        n3465 = Array Subset(array=w5430, index (col)=0 ("index"), length (col)=w5349) -> (w5435:dbl[][])  [unwired: 2 in]
        n3466 = Array Subset(array=w5430, index (col)=w5349) -> (w5433:dbl[][])  [unwired: 3 in]
        n3467 = for {
          tunnel: w5391 -> [w5482] mode=indexing
          tunnel: [w5481] -> w5390 mode=indexing
          workers-P: _ -> [_]
          n3468 = Reverse 1D Array(array=w5482) -> (reversed array=w5481:dbl[])
        }
        n3469 = for {
          tunnel: w5372 -> [w5480] mode=indexing
          tunnel: [w5479] -> w5371 mode=indexing
          workers-P: _ -> [_]
          n3470 = Reverse 1D Array(array=w5480) -> (reversed array=w5479:dbl[])
        }
        n3471 = for {
          tunnel: w5442 -> [w5488] mode=indexing
          tunnel: [w5487] -> w5441 mode=indexing
          workers-P: _ -> [_]
          n3472 = Reverse 1D Array(array=w5488) -> (reversed array=w5487:dbl[])
        }
        n3473 = for {
          tunnel: w5446 -> [w5490] mode=indexing
          tunnel: [w5489] -> w5445 mode=indexing
          workers-P: _ -> [_]
          n3474 = Reverse 1D Array(array=w5490) -> (reversed array=w5489:dbl[])
        }
        n3475 = for {
          tunnel: w5428 -> [w5484] mode=indexing
          tunnel: [w5483] -> w5427 mode=indexing
          workers-P: _ -> [_]
          n3476 = Reverse 1D Array(array=w5484) -> (reversed array=w5483:dbl[])
        }
        n3477 = for {
          tunnel: w5435 -> [w5486] mode=indexing
          tunnel: [w5485] -> w5434 mode=indexing
          workers-P: _ -> [_]
          n3478 = Reverse 1D Array(array=w5486) -> (reversed array=w5485:dbl[])
        }
        n3479 = Index Array(array=w5447, index (row)=0) -> (element=→"Waveform Graph":dbl[])  [unwired: 1 in]
        n3480 = Add(x=w5390, y=w5389) -> (x+y=w5382:dbl[][])
        n3481 = Add(x=w5371, y=w5370) -> (x+y=w5363:dbl[][])
        n3482 = Add(x=w5441, y=w5440) -> (x+y=w5439:dbl[][])
        n3483 = Add(x=w5445, y=w5444) -> (x+y=w5421:dbl[][])
        n3484 = Add(x=w5427, y=w5426) -> (x+y=w5425:dbl[][])
        n3485 = Add(x=w5434, y=w5433) -> (x+y=w5432:dbl[][])
        n3486 = Divide(x=w5425, y=2) -> (x/y=w5423:dbl[][])
        n3487 = Divide(x=w5439, y=2) -> (x/y=w5340:dbl[][])
        n3488 = To Single Precision Float(number=w5421) -> (single precision float=w5344:sgl[][])
        n3489 = To Single Precision Float(number=w5382) -> (single precision float=w5339:sgl[][])
        n3490 = To Single Precision Float(number=w5363) -> (single precision float=w5338:sgl[][])
        n3491 = Divide(x=w5432, y=2) -> (x/y=w5341:dbl[][])
        n3492 = Transpose 2D Array(2D array=w5423) -> (transposed array=→"Data map":dbl[][])
        n3493 = To Single Precision Float(number=w5340) -> (single precision float=w5343:sgl[][])
        n3494 = To Single Precision Float(number=w5341) -> (single precision float=w5342:sgl[][])
        n3495 = call "IMAQ ArrayToImage"("Image Pixels (Float)"=w5344, "Image"=w5380) -> ("Image Out"=→"APD 1":T8)  [unwired: 8 in, 1 out]
        n3496 = call "IMAQ ArrayToImage"("Image Pixels (Float)"=w5339, "Image"=w5379) -> ("Image Out"=→"APD 2":T8)  [unwired: 8 in, 1 out]
        n3497 = call "IMAQ ArrayToImage"("Image Pixels (Float)"=w5338, "Image"=w5360) -> ("Image Out"=→"APD 3":T8)  [unwired: 8 in, 1 out]
        n3498 = call "IMAQ ArrayToImage"("Image Pixels (Float)"=w5343, "Image"=w5361) -> ("Image Out"=→"Detection Laser X":T8)  [unwired: 8 in, 1 out]
        n3499 = call "IMAQ ArrayToImage"("Image Pixels (Float)"=w5342, "Image"=w5362) -> ("Image Out"=→"Detection Laser Y":T8)  [unwired: 8 in, 1 out]
      }
    }
    n3500 = case "For computing FFTs for display" shown="True" "Compute FFT" {
      tunnel: w4688 -> [_ w5687]
      frame False {
      }
      frame True {
        n3501 = Build Array("FFT 1 Choice 1", "FFT 1 Choice 2", "FFT 2 Choice 1", "FFT 2 Choice 2") -> (w5680:u16[])
        n3502 = Array Size(array=w5687) -> (size(s)=w5686:i32)
        n3503 = feedback-in #16(w5680) -> ()
        n3504 = feedback #16(u16[] [100, 100, 100, 100]) -> (w5681:u16[])
        n3505 = feedback-in #17("# Spectra to Ave.") -> ()
        n3506 = feedback #17("# Spectra to Ave.") -> (w5678:dbl)
        n3507 = Not Equal?(x="# Spectra to Ave.", y=w5678) -> (x != y?=w5677:bool)
        n3508 = Not Equal?(x=w5680, y=w5681) -> (x != y?=w5679:bool)
        n3509 = feedback #18(1.0) -> (w5664:dbl)
        n3510 = Compound Arithmetic op=OR("Reset FFT", w5679, w5677) -> (w5662:bool)
        n3511 = Select(t=1.0, s=w5662, f=w5664) -> (s? t:f=w5666:dbl)
        n3512 = Greater?(x=w5666, y="# Spectra to Ave.") -> (0:w5685:bool)
        n3513 = Increment(x=w5666) -> (x+1=w5665:dbl)
        n3514 = feedback-in #18(w5665) -> ()
        n3515 = local read "DMA Update Period (s)"() -> (w5660:dbl)
        n3516 = Multiply(x="# Spectra to Ave.", y=w5660) -> (x*y=→"Ave. Time (s)":dbl)
        n3517 = Build Array(cluster{"f0":dbl, "df":dbl, "magnitude":dbl[]} {"f0"=0.0, "df"=0.0, "magnitude"=[]} ("PSD")) -> (w5669:cluster{"f0":dbl, "df":dbl, "magnitude":dbl[]}[])
        n3518 = Build Array(w5669, w5669, w5669, w5669) -> (w5671:T73)
        n3519 = feedback #19(w5671) -> (w5676:T73)
        n3520 = for {
          N: 4 -> [_]
          tunnel: w5680 -> [w5709] mode=indexing
          tunnel: w5687 -> [w5710]
          tunnel: w5686 -> [w5712]
          tunnel: w5662 -> [w5705]
          tunnel: w5685 -> [w5704]
          tunnel: "# Spectra to Ave." -> [w5703]
          tunnel: [w5702] -> w5675 mode=indexing
          tunnel: w5676 -> [w5707] mode=indexing
          tunnel: [w5706] -> w5663 mode=indexing
          tunnel: w5666 -> [w5701]
          n3521 = Less?(x=w5709, y=w5712) -> (x < y?=w5711:bool)
          n3522 = Index Array(array=w5710, index=w5709) -> (element=w5708:waveform(dbl))
          n3523 = case shown="True" w5711 {
            tunnel: w5708 -> [_ w5729]
            tunnel: w5707 -> [w5714 w5727]
            tunnel: [w5714 w5715] -> w5706
            tunnel: w5705 -> [_ w5726]
            tunnel: w5704 -> [_ w5719]
            tunnel: w5703 -> [_ w5718]
            tunnel: [cluster{"f0":dbl, "df":dbl, "magnitude":dbl[]} {"f0"=0.0, "df"=0.0, "magnitude"=[]} ("PSD") w5720] -> w5702
            tunnel: w5701 -> [_ w5717]
            frame False {
            }
            frame True {
              n3524 = call <vilib>:"Std Deviation and Variance.vi"("X"=w5729) -> ("mean"=w5730:dbl)  [unwired: 1 in, 2 out]
              n3525 = Subtract(x=w5729, y=w5730) -> (x-y=w5728:waveform(dbl))
              n3526 = xnode "Spectral Measurements"("Signals"=w5728) -> ("PSD"=w5722:cluster{"f0":dbl, "df":dbl, "magnitude":dbl[]})  [unwired: 1 in, 1 out]
              n3527 = case shown="False" w5726 {
                tunnel: w5727 -> [w5739 _]
                tunnel: [w5735 w5744] -> w5715
                tunnel: w5722 -> [w5738 w5745]
                tunnel: w5719 -> [w5737 _]
                frame False {
                  n3528 = Build Array (concatenate)(w5739, w5738) -> (w5736:cluster{"f0":dbl, "df":dbl, "magnitude":dbl[]}[])
                  n3529 = case shown="True" w5737 {
                    tunnel: w5736 -> [w5740 w5743]
                    tunnel: [w5740 w5741] -> w5735
                    frame False {
                    }
                    frame True {
                      n3530 = Delete From Array(array=w5743, index=0) -> (array with subset deleted=w5741:cluster{"f0":dbl, "df":dbl, "magnitude":dbl[]}[])  [unwired: 1 in, 1 out]
                    }
                  }
                }
                frame True {
                  n3531 = Build Array(w5745) -> (w5744:cluster{"f0":dbl, "df":dbl, "magnitude":dbl[]}[])
                }
              }
              n3532 = for {
                tunnel: w5715 -> [w5734] mode=indexing
                tunnel: [w5733] -> w5725 mode=indexing
                workers-P: _ -> [_]
                n3533 = Unbundle By Name(w5734) -> ("magnitude"=w5733:dbl[])
              }
              n3534 = Transpose 2D Array(2D array=w5725) -> (transposed array=w5724:dbl[][])
              n3535 = for {
                tunnel: w5724 -> [w5732] mode=indexing
                tunnel: [w5731] -> w5723 mode=indexing
                workers-P: _ -> [_]
                n3536 = Add Array Elements(numeric array=w5732) -> (sum=w5731:dbl)
              }
              n3537 = Select(t=w5718, s=w5719, f=w5717) -> (s? t:f=w5716:dbl)
              n3538 = Divide(x=w5723, y=w5716) -> (x/y=w5721:dbl[])
              n3539 = Bundle By Name(cluster=w5722, "magnitude"=w5721) -> (w5720:cluster{"f0":dbl, "df":dbl, "magnitude":dbl[]})
            }
          }
        }
        n3540 = case shown="True" w5662 {
          tunnel: w5663 -> [w5694 w5700]
          tunnel: [w5694 w5695] -> w5661
          frame False {
          }
          frame True {
            n3541 = Array Subset(array=w5700, index (row)=0 ("index"), length (row)=4 ("length"), index (col)=0 ("index"), length (col)=1 ("length")) -> (w5695:T73)
          }
        }
        n3542 = feedback-in #19(w5661) -> ()
        n3543 = Split 1D Array(array=w5675, index=2) -> (first subarray=→"FFT 1":cluster{"f0":dbl, "df":dbl, "magnitude":dbl[]}[], second subarray=→"FFT 2":cluster{"f0":dbl, "df":dbl, "magnitude":dbl[]}[])
      }
    }
    n3544 = call-poly <vilib>:"Index Waveform Array.vi"("index"=16, "waveform array"=w4690) -> ("waveform"=w4713:waveform(dbl))  [unwired: 8 in, 1 out]
    n3545 = Unbundle By Name(w4713) -> ("Y"=→"PSD Y Sum":dbl[])
    n3546 = Not(x="Trap Trig. Fl.") -> (.not. x?=w4768:bool)
    n3547 = feedback-in #20("Trap Trig. Fl.") -> ()
    n3548 = feedback #20("Trap Trig. Fl.") -> (w4766:bool)
    n3549 = And(x=w4768, y=w4766) -> (x .and. y?=w4767:bool)
    n3550 = case "If have just turned off triggering" shown="True" w4767 {
      tunnel: w4706 -> [_ w5150]
      tunnel: w4762 -> [_ w5149]
      frame False {
      }
      frame True {
        w5148 = FALSE ("FPGA Trap Trig")
        n3551 = xnode "Read/Write Control"("FPGA VI Reference In"=w5150, "error in"=w5149, "FPGA Trap Trig"=w5148) -> ("FPGA VI Reference Out"=w5147:T40, "error out"=w5146:errorcluster)
        n3552 = xnode "Read/Write Control"("FPGA VI Reference In"=w5147, "error in"=w5146, "TTrig?"=w5148) -> ()  [unwired: 2 out]
        n3553 = local write "Initializing"(FALSE ("Initializing")) -> ()
        n3554 = local write "Triggered"(FALSE ("Triggered")) -> ()
        n3555 = local write "Waiting"(FALSE ("Waiting")) -> ()
      }
    }
    n3556 = Not(x=w4766) -> (.not. x?=w4779:bool)
    n3557 = And(x="Trap Trig. Fl.", y=w4779) -> (x .and. y?=w4776:bool)
    n3558 = local read "Tether"() -> (w4615:bool)
    n3559 = Or(x=w4776, y="Reinitialize") -> (x .or. y?=w4765:bool)
    n3560 = feedback #21(w4772) -> (w4777:string)
    n3561 = Select(t=w4772, s=w4776, f=w4777) -> (s? t:f=w4771:string)
    n3562 = Select(t=w4772, s="Reinitialize", f=w4771) -> (s? t:f=w4770:string)
    n3563 = feedback #22(0) -> (w4774:i32)
    n3564 = case "For determining if there is a tether still" shown="True" w4615 {
      tunnel: w4617 -> [_ w5259]
      frame False {
      }
      frame True {
        n3565 = Greater?(x="Lost Tether Alarm Threshold (pN)", y=w5259) -> (0:w5257:bool)
        n3566 = case shown="True" w5257 {
          frame False {
          }
          frame True {
            w5260 = FALSE ("Value (Signaling)")
            n3567 = flat-sequence {
              frame #0 {
                # "stop only if saving"
                n3568 = local read "Saving..."() -> (w5272:bool)
                n3569 = And(x=w5272, y="TA Cancel Save?") -> (x .and. y?=w5271:bool)
                n3570 = local write "Stop Saving"(w5271) -> ()
              }
              frame #1 {
                n3571 = case shown="True" "TA Green Off?" {
                  frame False {
                  }
                  frame True {
                    w5275 = FALSE ("Fl. Triggered...")
                    n3572 = local write "Fl. Triggered..."(w5275) -> ()
                    n3573 = property on="Green Laser ON" class="Bool (strict)"("Val(Sgnl)"=w5275) -> ()  [unwired: 2 in, 2 out]
                  }
                }
              }
            }
            n3574 = local read "Time tether formed"() -> (w5266:timestamp)
            n3575 = Get Date/Time In Seconds() -> (seconds since 1Jan1904=w5267:timestamp)
            n3576 = Subtract(x=w5267, y=w5266) -> (x-y=w5265:dbl)
            n3577 = Number To Decimal String(number=w5265) -> (decimal integer string=w5262:string)  [unwired: 1 out]
            n3578 = local read "Messages"() -> (w5269:string)
            n3579 = call <vilib>:"Beep.vi"() -> ()  [unwired: 3 in, 9 out]
            n3580 = Concatenate Strings("Lost tether (" ("Message to add"), w5262, " s)." ("string")) -> (w5264:string)
            n3581 = local write "Tether"(FALSE ("Tether")) -> ()
            n3582 = call "Update messages.vi"("Message to add"=w5264, "Old message string"=w5269) -> ("New message string"=w5268:string)
            n3583 = local write "Messages"(w5268) -> ()
            n3584 = property on="Fl. Triggered..." class="Bool (strict)"("Val(Sgnl)"=w5260) -> ()  [unwired: 2 in, 2 out]
            n3585 = local write "Dip for Protein"(w5260) -> ()
            n3586 = property on="Trap Pos. FB ON" class="Bool (strict)"("Val(Sgnl)"=w5260) -> ()  [unwired: 2 in, 2 out]
            n3587 = property on="Trap Trig. Fl." class="Bool (strict)"("Val(Sgnl)"=w5260) -> ()  [unwired: 2 in, 2 out]
          }
        }
      }
    }
    n3588 = case "For triggering actions based on the trap position (e.g., turning the excitation laser on if trap under feedback moves so far)" shown="True" "Trap Trig. Fl." {
      tunnel: w4654 -> [_ w5163]
      tunnel: w4770 -> [_ w5162]
      tunnel: ["" ("t") w5161] -> w4778
      tunnel: w4765 -> [_ w5160]
      tunnel: [0 ("t") w5159] -> w4775
      tunnel: w4774 -> [_ w5158]
      tunnel: w4706 -> [_ w5157]
      tunnel: w4762 -> [_ w5156]
      frame False {
      }
      frame True {
        n3589 = case shown="\"Wait for trigger\"" w5162 {
          tunnel: w5163 -> [w5180 _ _ w5228]
          tunnel: [w5177 w5209 "" ("t") w5231] -> w5161
          tunnel: w5160 -> [_ _ _ w5219]
          tunnel: [w5176 w5206 0 ("t") w5220] -> w5159
          tunnel: w5158 -> [_ w5208 _ w5226]
          tunnel: w5157 -> [w5165 w5203 _ w5222]
          tunnel: w5156 -> [w5164 w5202 _ w5221]
          frame "Wait for trigger" {
            n3590 = local read "Trap Trig. (FPGA)"() -> (w5168:bool)
            n3591 = Subtract(x=w5180, y="Mean T1 Position\nto compare (nm)") -> (x-y=w5173:dbl[])
            n3592 = call <vilib>:"Std Deviation and Variance.vi"("X"=w5173) -> ("mean"=→"mean":dbl, "standard deviation"=→"standard\ndeviation":dbl)  [unwired: 1 in, 1 out]
            n3593 = Array Max & Min(array=w5173) -> (max value=→"max value":dbl, min value=→"min value":dbl)  [unwired: 2 out]
            n3594 = Greater?(x=w5173, y="Threshold (nm)") -> (0:w5183:bool[])
            n3595 = case shown="True" w5168 {
              tunnel: w5165 -> [_ w5189]
              tunnel: w5164 -> [_ w5188]
              tunnel: [FALSE ("TTrig?") w5187] -> w5171
              frame False {
              }
              frame True {
                n3596 = xnode "Read/Write Control"("FPGA VI Reference In"=w5189, "error in"=w5188) -> ("TTrig?"=w5187:bool)  [unwired: 2 out]
              }
            }
            n3597 = Or Array Elements(Boolean array=w5183) -> (logical OR=w5170:bool)
            n3598 = Select(t=w5171, s=w5168, f=w5170) -> (s? t:f=w5169:bool)
            n3599 = Not(x=w5168) -> (.not. x?=w5167:bool)
            n3600 = And(x=w5169, y=w5167) -> (x .and. y?=w5166:bool)
            n3601 = Select(t="Triggered", s=w5169, f="Wait for trigger") -> (s? t:f=w5177:string)
            n3602 = case shown="True" w5169 {
              tunnel: [0 0] -> w5176
              tunnel: w5165 -> [_ w5194]
              tunnel: w5164 -> [_ w5193]
              frame False {
                "Waiting" <- TRUE ("Waiting")
              }
              frame True {
                n3603 = xnode "Read/Write Control"("FPGA VI Reference In"=w5194, "error in"=w5193, "TTrig?"=FALSE) -> ()  [unwired: 2 out]
                n3604 = local read "Messages"() -> (w5197:string)
                n3605 = call <vilib>:"Beep.vi"() -> ()  [unwired: 12 in]
                n3606 = call "Update messages.vi"("Message to add"="Unwinding trigger.", "Old message string"=w5197) -> ("New message string"=w5198:string)
                n3607 = local write "Messages"(w5198) -> ()
                n3608 = local write "Waiting"(FALSE ("Waiting")) -> ()
                "Triggered" <- TRUE ("Triggered")
              }
            }
            n3609 = case "Only need to turn on laser if host triggered" shown="True" w5166 {
              frame False {
              }
              frame True {
                n3610 = property on="Green Laser ON" class="Bool (strict)"("Val(Sgnl)"=TRUE ("Value (Signaling)")) -> ()  [unwired: 2 in, 2 out]
              }
            }
          }
          frame "Triggered" {
            n3611 = local read "Trap Trig. (FPGA)"() -> (w5205:bool)
            n3612 = Increment(x=w5208) -> (x+1=w5206:i32)
            n3613 = Greater Or Equal?(x=w5206, y="Fl. ON time (n)") -> (x >= y?=w5204:bool)
            n3614 = Select(t="Wait for trigger", s=w5204, f="Triggered" ("t")) -> (s? t:f=w5209:string)
            n3615 = And(x=w5204, y=w5205) -> (x .and. y?=w5201:bool)
            n3616 = case shown="True" w5201 {
              tunnel: w5203 -> [_ w5213]